vi "UHR-Fleezers Control (host) - 12.7b.vi"() -> ()   [LabVIEW 2012] (continued)
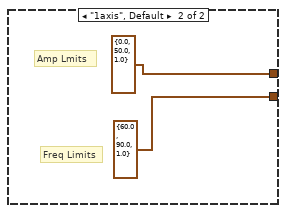
[diagram p2: hidden frame]
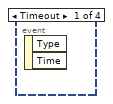
[diagram p3: hidden frame]
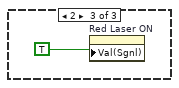
[diagram p6: hidden frame]
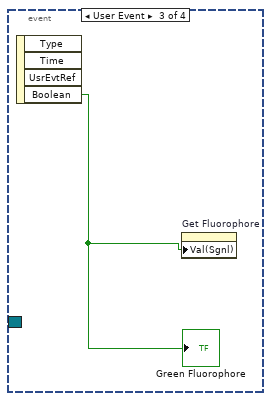
[diagram p7: hidden frame]
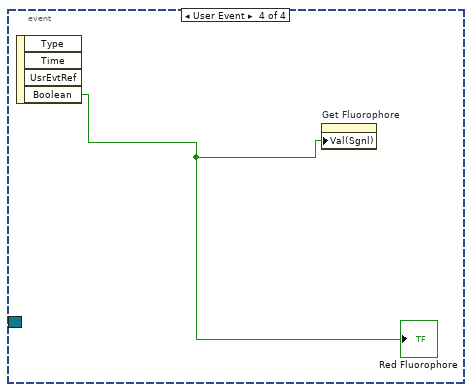
[diagram p8: hidden frame]
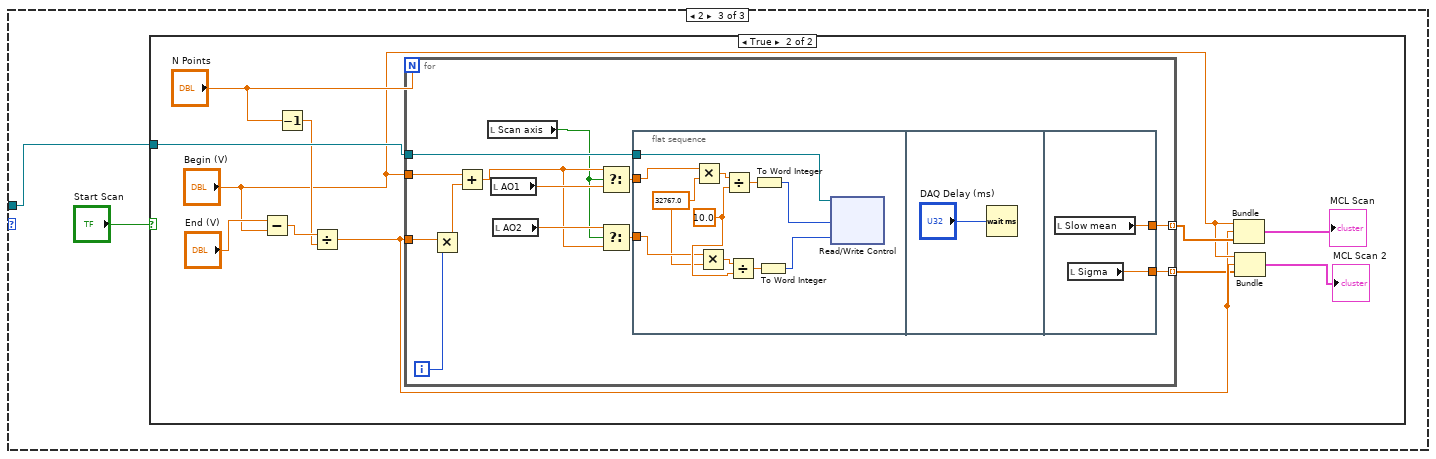
[diagram p10: hidden frame]
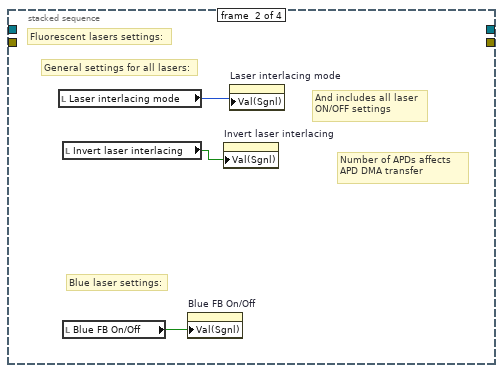
[diagram p12: hidden frame]
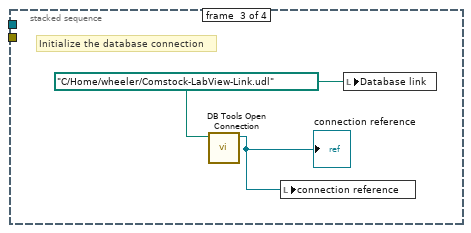
[diagram p13: hidden frame]
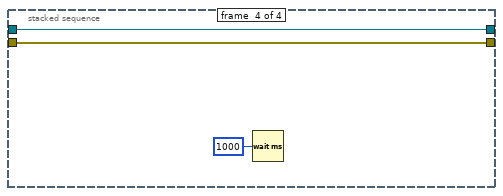
[diagram p14: hidden frame]
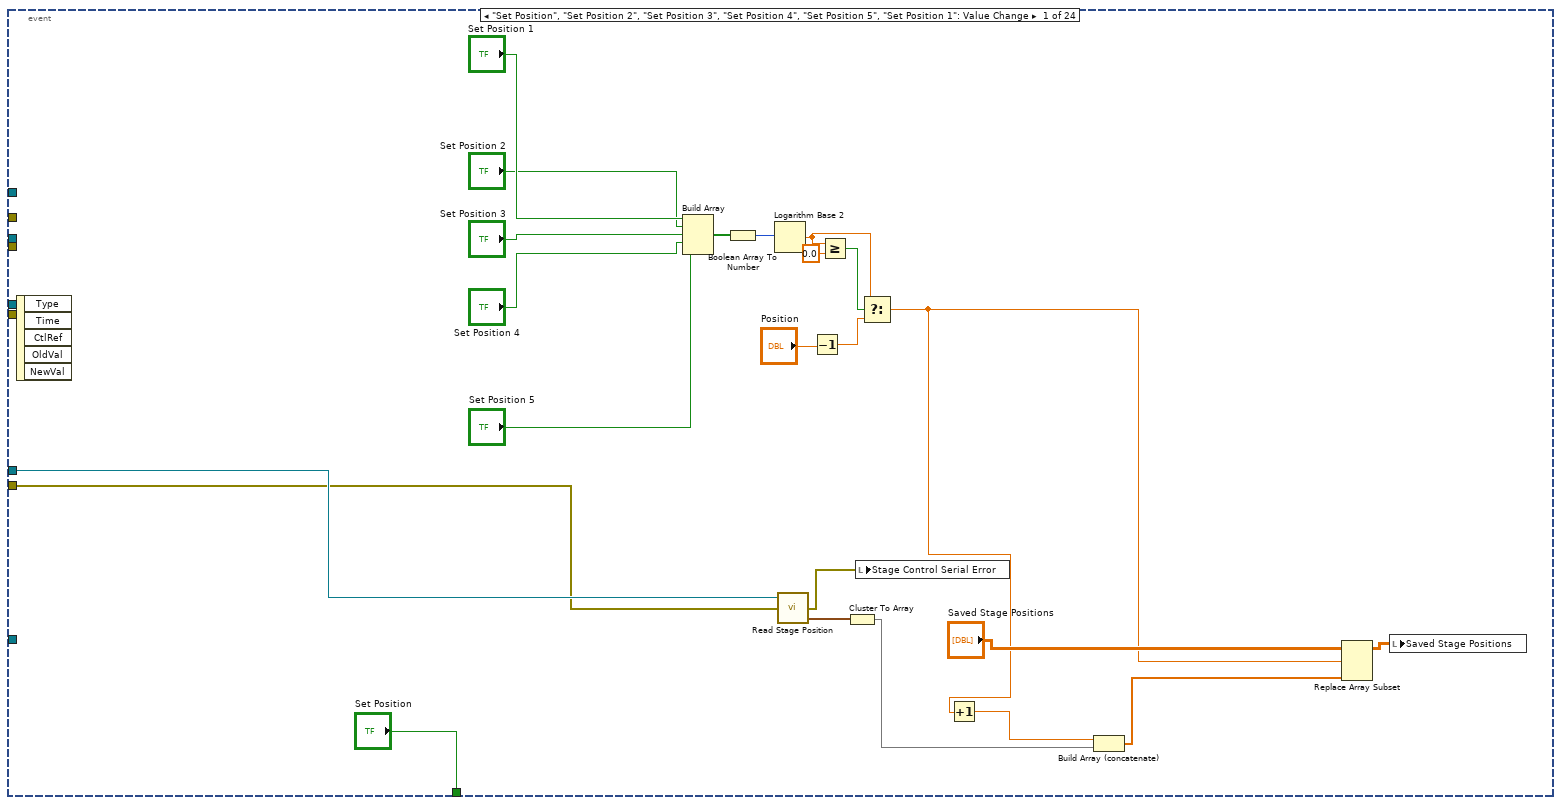
[diagram p16: hidden frame]
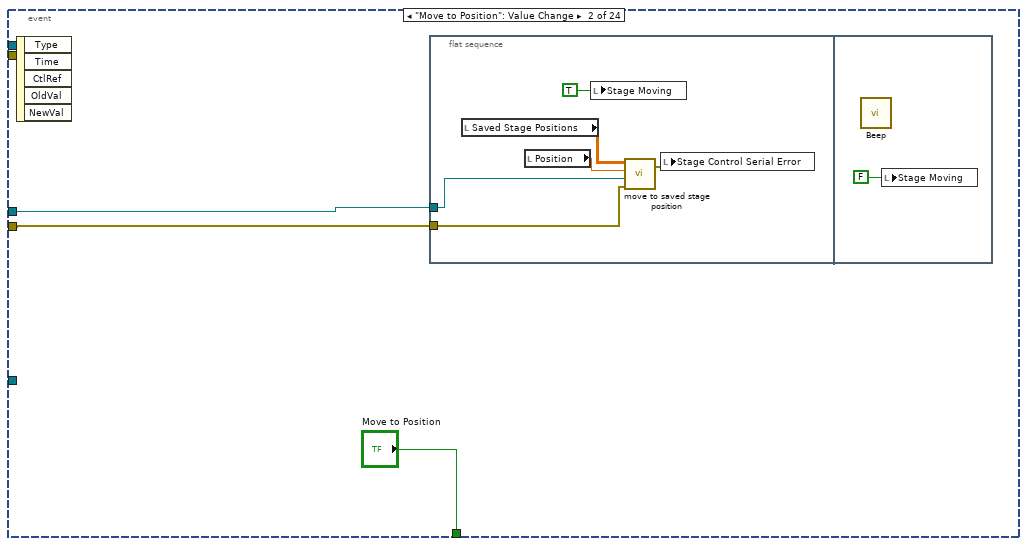
[diagram p17: hidden frame]
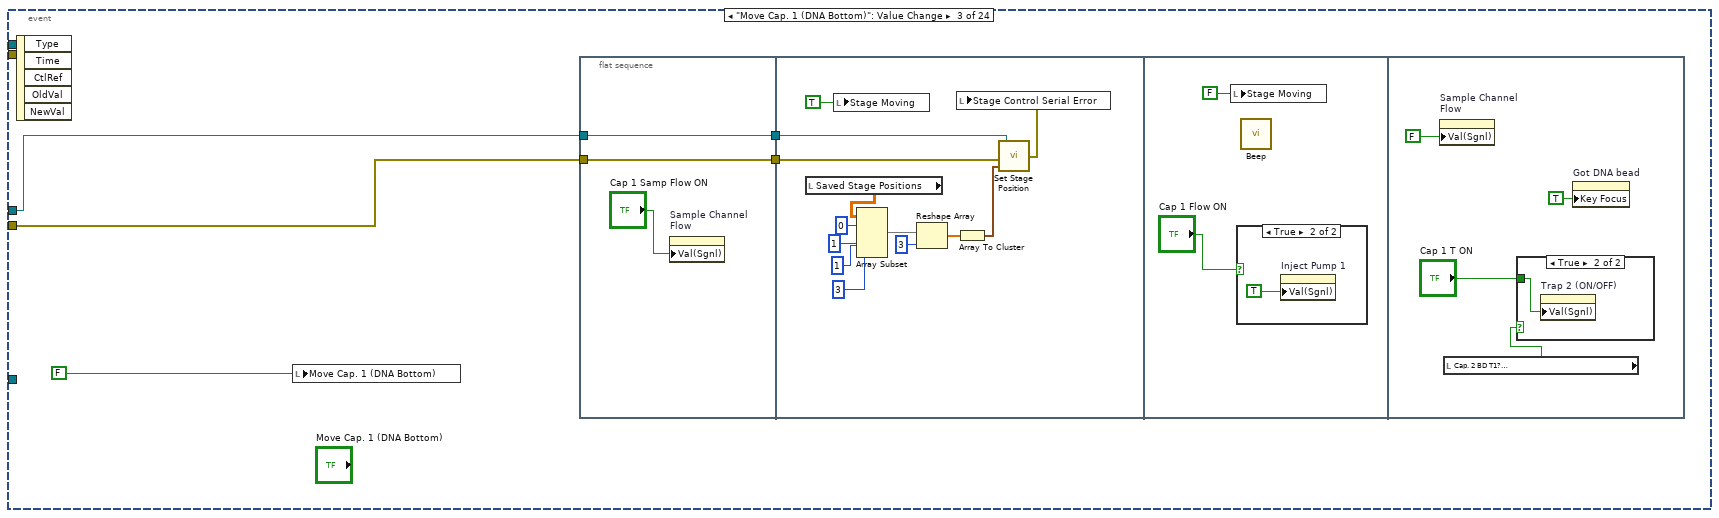
[diagram p18: hidden frame]
                n3006 = Build Array (concatenate)(w4814, w4813, w4806) -> (w4812:dbl[])
                "Calibrating Trap..." <- TRUE ("Calibrating...")
              }
              frame 4 {
                w4824 = 0.0 ("f")
                # "scan dir (x/y = 0/1)"
                # "cycles/step"
                # "n scans (f/b)"
                # "steps"
                # "freq. range"
                # "AOD raster scan"
                n3007 = local read "Number of F/B Scans (AOD)"() -> (w4831:u16)
                n3008 = local read "Cycles/step (AOD)"() -> (w4833:u64)
                n3009 = local read "Scan Range (MHz)"() -> (w4836:dbl)
                n3010 = local read "Scan steps (AOD)"() -> (w4835:u64)
                n3011 = local read "Scan BD"() -> (w4843:bool)
                n3012 = local read "Save ave N"() -> (w4848:dbl)
                n3013 = Boolean To (0,1)(Boolean=w4843) -> (0, 1=w4842:i16)
                n3014 = To Double Precision Float(number=w4831) -> (double precision float=w4830:dbl)
                n3015 = To Double Precision Float(number=w4835) -> (double precision float=w4834:dbl)
                n3016 = To Double Precision Float(number=w4833) -> (double precision float=w4832:dbl)
                n3017 = To Double Precision Float(number=w4842) -> (double precision float=w4841:dbl)
                n3018 = Multiply(x=w4848, y=w4826) -> (x*y=w4847:dbl)
                n3019 = To Double Precision Float(number=w4819) -> (double precision float=w4825:dbl)
                n3020 = Build Array(w4825, w4824, w4824, w4824, w4824) -> (w4822:dbl[])
                n3021 = local read "N sets should be saved"() -> (w4828:dbl)
                n3022 = Build Array(w4841, w4836, w4834, w4832, w4830) -> (w4838:dbl[])
                n3023 = Build Array(w4821, w4826, w4847, w4846, w4845, 2.0 ("t")) -> (w4840:dbl[])
                n3024 = Round Toward +Infinity(x=w4828) -> (ceil(x): smallest int >= x=w4829:dbl)
                n3025 = Build Array (concatenate)(w4840, w4839, w4822, w4838) -> (w4837:dbl[])
                n3026 = To Unsigned Long Integer(number=w4829) -> (unsigned 32bit integer=w4827:u32)
              }
              frame 8 {
                w4857 = 0.0 ("f")
                # "MCL raster scan"
                n3027 = local read "Number of scans (MCL)"() -> (w4852:u64)
                n3028 = local read "Scan lines (y)"() -> (w4851:u64)
                n3029 = local read "2D or 1D Scan"() -> (w4854:bool)
                n3030 = local read "Scan Range (V)\n(of steps)"() -> (w4873:dbl)
                n3031 = local read "Fast Scan Dir"() -> (w4880:bool)
                n3032 = local read "Cycles/step (MCL)"() -> (w4870:u64)
                n3033 = local read "Scan steps (MCL)"() -> (w4872:u64)
                n3034 = Select(t=w4851, s=w4854, f=w4852) -> (s? t:f=w4853:u64)
                n3035 = Boolean To (0,1)(Boolean=w4854) -> (0, 1=w4856:i16)
                n3036 = local read "Save ave N"() -> (w4885:dbl)
                n3037 = local read "Initial X"() -> (w4859:dbl)
                n3038 = local read "Initial Y"() -> (w4858:dbl)
                n3039 = To Double Precision Float(number=w4856) -> (double precision float=w4855:dbl)
                n3040 = Boolean To (0,1)(Boolean=w4880) -> (0, 1=w4879:i16)
                n3041 = To Double Precision Float(number=w4853) -> (double precision float=w4868:dbl)
                n3042 = To Double Precision Float(number=w4872) -> (double precision float=w4871:dbl)
                n3043 = To Double Precision Float(number=w4870) -> (double precision float=w4869:dbl)
                n3044 = To Double Precision Float(number=w4879) -> (double precision float=w4878:dbl)
                n3045 = Multiply(x=w4885, y=w4864) -> (x*y=w4884:dbl)
                n3046 = To Double Precision Float(number=w4849) -> (double precision float=w4863:dbl)
                n3047 = local read "N sets should be saved (MCL)"() -> (w4866:dbl)
                n3048 = Build Array(w4863, w4855, w4857, w4857, w4857) -> (w4861:dbl[])
                n3049 = Build Array(w4878, w4873, w4871, w4869, w4868, w4859, w4858) -> (w4875:dbl[])
                n3050 = Build Array(w4860, w4864, w4884, w4883, w4882, 3.0 ("t")) -> (w4877:dbl[])
                n3051 = Round Toward +Infinity(x=w4866) -> (ceil(x): smallest int >= x=w4867:dbl)
                n3052 = Build Array (concatenate)(w4877, w4876, w4861, w4875) -> (w4874:dbl[])
                n3053 = To Unsigned Long Integer(number=w4867) -> (unsigned 32bit integer=w4865:u32)
              }
            }
            n3054 = local read "Index"() -> (w4723:dbl)
            n3055 = call "Create new save file.vi"("Insert"="", "Ext"=".dat", "Index In"=w4723) -> ("Path Out"=w4679:path, "Index Out"=w4697:dbl)
            n3056 = local write "Save file name"(w4679) -> ()
            n3057 = local write "Index"(w4697) -> ()
            n3058 = local write "Save index"(w4697) -> ()
            n3059 = Array Size(array=w4706) -> (size(s)=w4707:i32)
            n3060 = Open/Create/Replace File(file path (use dialog)=w4679, operation (0:open)=T29."create", access (0:read/write)=enum16{"read/write", "read-only", "write-only"}."write-only") -> (refnum out=w4720:refnum<file>)  [unwired: 1 in, 4 out]
            n3061 = local write "Saving..."(TRUE ("Saving...")) -> ()
            n3062 = To Double Precision Float(number=w4707) -> (double precision float=w4705:dbl)
            n3063 = String Length(string="Comment (data description)") -> (length=w4704:i32)
            n3064 = To Double Precision Float(number=w4704) -> (double precision float=w4703:dbl)
            n3065 = Deny Access(7:w4720) -> (3:w4719:refnum<file>)  [unwired: 1 in, 2 out]
            n3066 = Build Array (concatenate)(w4705, w4706, w4703) -> (w4678:dbl[])
            n3067 = case "If fluorescence data to be saved" shown="True" w4695 {
              tunnel: w4679 -> [_ w4773]
              tunnel: [refnum<k0> refnum w4753] -> w4696
              frame False {
              }
              frame True {
                w4752 = 0.0
                n3068 = local read "APD Integration Time (s)"() -> (w4758:dbl)
                n3069 = local read "N APD Samp/step"() -> (w4751:dbl)
                n3070 = local read "Number of APDs"() -> (w4750:u8)
                n3071 = Path To String(path=w4773) -> (string=w4772:string)
                n3072 = String Length(string=w4772) -> (length=w4771:i32)
                n3073 = Subtract(x=w4771, y=4) -> (x-y=w4769:i32)
                n3074 = String Subset(string=w4772, length (rest)=w4769) -> (substring=w4768:string)  [unwired: 1 out]
                n3075 = Build Array(w4758, w4751, w4750, w4752, w4752, w4752, w4752, w4752) -> (w4755:dbl[])
                n3076 = Concatenate Strings(w4768, "_fl.dat" ("string")) -> (w4766:string)
                n3077 = Array Size(array=w4755) -> (size(s)=w4757:i32)
                n3078 = String To Path(string=w4766) -> (path=w4762:path)
                n3079 = Open/Create/Replace File(file path (use dialog)=w4762, operation (0:open)=T29."create", access (0:read/write)=enum16{"read/write", "read-only", "write-only"}."write-only") -> (refnum out=w4763:refnum<file>)  [unwired: 1 in, 4 out]
                n3080 = Deny Access(7:w4763) -> (3:w4759:refnum<file>)  [unwired: 1 in, 2 out]
                n3081 = To Double Precision Float(number=w4757) -> (double precision float=w4756:dbl)
                n3082 = Build Array (concatenate)(w4756, w4755) -> (w4754:dbl[])
                n3083 = Write to Binary File(file (use dialog)=w4759, data=w4754, 5:FALSE ("prepend array or string size? (T)"), 9:T28."big-endian, network order" ("byte order (0:big-endian, network order)")) -> (refnum out=w4753:refnum<file>)  [unwired: 1 in, 3 out]
              }
            }
            n3084 = case shown="True" w4683 {
              tunnel: w4679 -> [_ w4734]
              tunnel: [refnum<k0> refnum w4733] -> w4684
              frame False {
              }
              frame True {
                w4729 = 0.0 ("element")
                n3085 = Path To String(path=w4734) -> (string=w4748:string)
                n3086 = Build Array(w4729, w4729, w4729, w4729, w4729, w4729, w4729, w4729) -> (w4730:dbl[])
                n3087 = String Length(string=w4748) -> (length=w4747:i32)
                n3088 = Subtract(x=w4747, y=4) -> (x-y=w4745:i32)
                n3089 = Array Size(array=w4730) -> (size(s)=w4732:i32)
                n3090 = String Subset(string=w4748, length (rest)=w4745) -> (substring=w4744:string)  [unwired: 1 out]
                n3091 = To Double Precision Float(number=w4732) -> (double precision float=w4731:dbl)
                n3092 = Concatenate Strings(w4744, "_pos.dat" ("string")) -> (w4742:string)
                n3093 = Build Array (concatenate)(w4731, w4730) -> (w4728:dbl[])
                n3094 = String To Path(string=w4742) -> (path=w4738:path)
                n3095 = Open/Create/Replace File(file path (use dialog)=w4738, operation (0:open)=T29."create", access (0:read/write)=enum16{"read/write", "read-only", "write-only"}."write-only") -> (refnum out=w4739:refnum<file>)  [unwired: 1 in, 4 out]
                n3096 = Deny Access(7:w4739) -> (3:w4735:refnum<file>)  [unwired: 1 in, 2 out]
                n3097 = Write to Binary File(file (use dialog)=w4735, data=w4728, 5:FALSE ("prepend array or string size? (T)"), 9:T28."big-endian, network order" ("byte order (0:big-endian, network order)")) -> (refnum out=w4733:refnum<file>)  [unwired: 1 in, 3 out]
              }
            }
            n3098 = Write to Binary File(file (use dialog)=w4719, data=w4678, 5:w4701, 9:w4700) -> (refnum out=w4702:refnum<file>)  [unwired: 1 in, 3 out]
            n3099 = Write to Binary File(file (use dialog)=w4702, data="Comment (data description)", 5:w4701, 9:w4700) -> (refnum out=w4699:refnum<file>)  [unwired: 1 in, 3 out]
            n3100 = local read "connection reference"() -> (w4681:T17)
            n3101 = Bundle("Comment (data description)"="Comment (data description)", "Channel 1 Buffer"="Channel 1 Buffer", "Channel 2 Buffer"="Channel 2 Buffer", "Channel 3 Buffer"="Channel 3 Buffer", "Title"="Title", "DNA Construct"="DNA Construct", "Bead diameter"="Bead diameter", "Name"="Name") -> (w4669:T47)  [unwired: 1 in]
            n3102 = call "MattFileCreator-v9.vi"("Comments"=w4669, "Input Array"=w4678, "File path"=w4679, "table"="labview", "connection reference"=w4681) -> ("connection reference out"=w4680:T17)  [unwired: 5 in, 1 out]
            n3103 = local write "connection reference"(w4680) -> ()
          }
        }
        n3104 = feedback-in #27(w4629) -> ()
        n3105 = feedback-in #28(w4656) -> ()
        n3106 = feedback-in #29(w4628) -> ()
        n3107 = feedback-in #30(w4639) -> ()
        n3108 = feedback-in #31(w4642) -> ()
        n3109 = feedback-in #32(w4655) -> ()
        n3110 = feedback-in #33(w4645) -> ()
      }
      frame #1 {
        n3111 = local read "Saving..."() -> (w4899:bool)
        n3112 = case shown="True" w4899 {
          tunnel: w4903 -> [_ w4914]
          tunnel: w4902 -> [_ w4928]
          tunnel: w4901 -> [_ w4924]
          tunnel: w4900 -> [_ w4923]
          tunnel: w4898 -> [_ w4922]
          tunnel: w4897 -> [_ w4917]
          tunnel: w4896 -> [_ w4916]
          tunnel: w4895 -> [_ w4915]
          tunnel: w4894 -> [_ w4913]
          tunnel: w4893 -> [_ w4911]
          tunnel: w4892 -> [_ w4910]
          tunnel: w4891 -> [_ w4909]
          tunnel: w4890 -> [_ w4908]
          tunnel: w4889 -> [_ w4907]
          tunnel: w4888 -> [_ w4906]
          tunnel: w4887 -> [_ w4905]
          tunnel: w4886 -> [_ w4904]
          frame False {
          }
          frame True {
            n3113 = Multiply(x=w4914, y=w4913) -> (x*y=→"Time (s)":dbl)
            n3114 = Less Or Equal?(x=w4914, y=w4922) -> (x <= y?=w4926:bool)
            n3115 = Or(x="Stop Saving", y="Abort save 2") -> (x .or. y?=w4918:bool)
            n3116 = Not(x=w4918) -> (.not. x?=w4927:bool)
            n3117 = And(x=w4926, y=w4927) -> (x .and. y?=w4925:bool)
            n3118 = case shown="True" w4925 {
              tunnel: w4928 -> [w4935 w5026]
              tunnel: [0.0 w5029] -> w4921
              tunnel: w4914 -> [_ w5027]
              tunnel: w4922 -> [_ w5028]
              tunnel: w4924 -> [_ w5023]
              tunnel: w4923 -> [_ _]
              tunnel: w4917 -> [w4933 w5016]
              tunnel: w4916 -> [w4932 w5017]
              tunnel: w4915 -> [_ w5015]
              tunnel: w4911 -> [_ w5014]
              tunnel: w4910 -> [_ w4938]
              tunnel: w4909 -> [_ w5007]
              tunnel: w4908 -> [_ w4954]
              tunnel: w4907 -> [w4929 w4971]
              tunnel: w4906 -> [w4930 w4970]
              tunnel: w4905 -> [_ w4967]
              tunnel: w4904 -> [_ w4965]
              frame False {
                w4931 = FALSE
                n3119 = Close File(refnum=w4935) -> ()  [unwired: 1 in, 2 out]
                n3120 = case shown="True" w4932 {
                  tunnel: w4933 -> [_ w4937]
                  frame False {
                  }
                  frame True {
                    n3121 = Close File(refnum=w4937) -> ()  [unwired: 1 in, 2 out]
                  }
                }
                n3122 = case shown="True" w4929 {
                  tunnel: w4930 -> [_ w4936]
                  frame False {
                  }
                  frame True {
                    n3123 = Close File(refnum=w4936) -> ()  [unwired: 1 in, 2 out]
                  }
                }
                n3124 = local write "Raster Scanning..."(w4931) -> ()
                n3125 = local write "Calibrating Trap..."(w4931) -> ()
                n3126 = call <vilib>:"Beep.vi"() -> ()  [unwired: 3 in, 9 out]
                n3127 = local write "Stop Saving"(w4931) -> ()
                "Saving..." <- w4931
              }
              frame True {
                n3128 = local read "Calibrating Trap..."() -> (w5018:bool)
                n3129 = case "Write fl. data" shown="True" w5017 {
                  tunnel: w5016 -> [_ w5052]
                  tunnel: w5015 -> [_ w5051]
                  frame False {
                  }
                  frame True {
                    n3130 = Write to Binary File(file (use dialog)=w5052, data=w5051, 5:FALSE ("prepend array or string size? (T)"), 9:T28."big-endian, network order" ("byte order (0:big-endian, network order)")) -> ()  [unwired: 1 in, 4 out]
                  }
                }
                n3131 = Greater?(x="Save ave N", y=1.0) -> (0:w5021:bool)
                n3132 = Not(x=w5018) -> (.not. x?=w5020:bool)
                n3133 = And(x=w5020, y=w5021) -> (x .and. y?=w4968:bool)
                n3134 = case shown="True" w4968 {
                  tunnel: w4967 -> [w5032 w5043]
                  tunnel: [w5032 w5035] -> w4966
                  tunnel: "Save ave N" -> [_ w5036]
                  frame False {
                  }
                  frame True {
                    w5033 = 2 ("dimension size")
                    n3135 = Array Size(array=w5043) -> (size(s)=w5037:i32)
                    n3136 = Divide(x=w5037, y=w5033) -> (x/y=w5041:dbl)
                    n3137 = Reshape Array(w5043, w5041, w5033) -> (w5042:u64[][])
                    n3138 = Transpose 2D Array(2D array=w5042) -> (transposed array=w5040:u64[][])
                    n3139 = for {
                      tunnel: w5040 -> [w5045] mode=indexing
                      tunnel: [w5044] -> w5034 mode=indexing
                      tunnel: w5036 -> [w5046]
                      workers-P: _ -> [_]
                      n3140 = call "downsample 1D array - U64.vi"("Ave N"=w5046, "Array In"=w5045) -> ("Array Out"=w5044:u64[])  [unwired: 1 in]
                    }
                    n3141 = Transpose 2D Array(2D array=w5034) -> (transposed array=w5039:u64[][])
                    n3142 = Divide(x=w5037, y=w5036) -> (x/y=w5038:dbl)
                    n3143 = Reshape Array(w5039, w5038) -> (w5035:u64[])
                  }
                }
                n3144 = case shown="True" w4968 {
                  tunnel: w5023 -> [w5055 w5067]
                  tunnel: [w5055 w5059] -> w5019
                  tunnel: "Save ave N" -> [_ w5060]
                  tunnel: w5014 -> [_ w5058]
                  frame False {
                  }
                  frame True {
                    n3145 = Array Size(array=w5067) -> (size(s)=w5061:i32)
                    n3146 = Array Size(array=w5058) -> (size(s)=w5057:i32)
                    n3147 = Divide(x=w5061, y=w5057) -> (x/y=w5065:dbl)
                    n3148 = Reshape Array(w5067, w5065, w5057) -> (w5066:i16[][])
                    n3149 = Transpose 2D Array(2D array=w5066) -> (transposed array=w5064:i16[][])
                    n3150 = for {
                      tunnel: w5064 -> [w5070] mode=indexing
                      tunnel: [w5069] -> w5056 mode=indexing
                      tunnel: w5060 -> [w5068]
                      workers-P: _ -> [_]
                      n3151 = call "downsample 1D array - I16.vi"("Ave N"=w5068, "Array In"=w5070) -> ("Array Out"=w5069:i16[])  [unwired: 1 out]
                    }
                    n3152 = Transpose 2D Array(2D array=w5056) -> (transposed array=w5063:i16[][])
                    n3153 = Divide(x=w5061, y=w5060) -> (x/y=w5062:dbl)
                    n3154 = Reshape Array(w5063, w5062) -> (w5059:i16[])
                  }
                }
                n3155 = Index Array(array=w4954, index=2) -> (element=w4955:waveform(dbl))
                n3156 = Index Array(array=w4954, index=1) -> (element=w4988:waveform(dbl))
                n3157 = Index Array(array=w4954, index=0) -> (element=w4990:waveform(dbl))
                n3158 = Unbundle By Name(w4955) -> ("Y"=w4957:dbl[])
                n3159 = Unbundle By Name(w4988) -> ("Y"=w4992:dbl[])
                n3160 = Unbundle By Name(w4990) -> ("Y"=w5000:dbl[])
                n3161 = case "Write trap pos. data" shown="True" w4971 {
                  tunnel: w4970 -> [_ w5048]
                  tunnel: w4966 -> [_ w5047]
                  frame False {
                  }
                  frame True {
                    n3162 = Write to Binary File(file (use dialog)=w5048, data=w5047, 5:FALSE ("prepend array or string size? (T)"), 9:T28."big-endian, network order" ("byte order (0:big-endian, network order)")) -> ()  [unwired: 1 in, 4 out]
                  }
                }
                n3163 = Write to Binary File(file (use dialog)=w5026, data=w5019, 5:FALSE ("prepend array or string size? (T)"), 9:T28."big-endian, network order" ("byte order (0:big-endian, network order)")) -> ()  [unwired: 1 in, 4 out]
                n3164 = feedback #34(w4957) -> (w4958:dbl[])
                n3165 = Build Array (concatenate)(w4958, w4957) -> (w4953:dbl[])
                n3166 = Select(t=w4957, s=w4938, f=w4953) -> (s? t:f=w4943:dbl[])
                n3167 = feedback-in #34(w4943) -> ()
                n3168 = feedback #35(w4992) -> (w4994:dbl[])
                n3169 = Build Array (concatenate)(w4994, w4992) -> (w4993:dbl[])
                n3170 = Select(t=w4992, s=w4938, f=w4993) -> (s? t:f=w4982:dbl[])
                n3171 = feedback-in #35(w4982) -> ()
                n3172 = feedback #36(w5000) -> (w5013:dbl[])
                n3173 = Build Array (concatenate)(w5013, w5000) -> (w5012:dbl[])
                n3174 = Select(t=w5000, s=w4938, f=w5012) -> (s? t:f=w4987:dbl[])
                n3175 = feedback-in #36(w4987) -> ()
                n3176 = Divide(x=w5027, y=w5028) -> (x/y=w5030:dbl)
                n3177 = Multiply(x=w5030, y=100.0) -> (x*y=w5029:dbl)
                n3178 = Build Array(w4987, w4982, w4943) -> (→"Saved APD":dbl[][])
                n3179 = Array Size(array=w4987) -> (size(s)=w5005:i32)
                n3180 = Unbundle By Name(w5007) -> ("Y"=w5011:dbl[])
                n3181 = Subtract(x=w5005, y="N pts to average") -> (x-y=w4940:i32)
                n3182 = Multiply(x="N pts to average", y=u16 2) -> (x*y=w4983:u16)
                n3183 = Subtract(x=w5005, y=w4983) -> (x-y=w4941:i32)
                n3184 = feedback #37(w5011) -> (w5010:dbl[])
                n3185 = Build Array (concatenate)(w5010, w5011) -> (w5009:dbl[])
                n3186 = Select(t=w5011, s=w4938, f=w5009) -> (s? t:f=w5008:dbl[])
                "Trap Delta Graph" <- w5008
                n3187 = feedback-in #37(w5008) -> ()
                n3188 = Array Subset(array=w4987, index=w4940, length="N pts to average") -> (w5004:dbl[])
                n3189 = Array Subset(array=w4987, index=w4941, length="N pts to average") -> (w5003:dbl[])
                n3190 = Array Subset(array=w4982, index=w4940, length="N pts to average") -> (w4985:dbl[])
                n3191 = Array Subset(array=w4982, index=w4941, length="N pts to average") -> (w4984:dbl[])
                n3192 = Array Subset(array=w4943, index=w4940, length="N pts to average") -> (w4952:dbl[])
                n3193 = Array Subset(array=w4943, index=w4941, length="N pts to average") -> (w4951:dbl[])
                n3194 = Index Array(array=w4965, index=0) -> (element=w4963:waveform(dbl))
                n3195 = call-poly <vilib>:"Mean.vi"("X"=w5004) -> ("mean"=w5002:dbl)  [unwired: 1 out]
                n3196 = call-poly <vilib>:"Mean.vi"("X"=w4985) -> ("mean"=w4981:dbl)  [unwired: 1 out]
                n3197 = call-poly <vilib>:"Mean.vi"("X"=w5003) -> ("mean"=w5001:dbl)  [unwired: 1 out]
                n3198 = call-poly <vilib>:"Mean.vi"("X"=w4984) -> ("mean"=w4980:dbl)  [unwired: 1 out]
                n3199 = call-poly <vilib>:"Mean.vi"("X"=w4952) -> ("mean"=w4950:dbl)  [unwired: 1 out]
                n3200 = call-poly <vilib>:"Mean.vi"("X"=w4951) -> ("mean"=w4949:dbl)  [unwired: 1 out]
                n3201 = Unbundle By Name(w4963) -> ("Y"=w4961:dbl[])
                n3202 = Subtract(x=w4981, y=w4980) -> (x-y=w4972:dbl)
                "Delta Fl. 2" <- w4972
                n3203 = Subtract(x=w4950, y=w4949) -> (x-y=w4944:dbl)
                "Delta Fl. 3" <- w4944
                n3204 = Subtract(x=w5002, y=w5001) -> (x-y=w4999:dbl)
                "Delta Fl. 1" <- w4999
                n3205 = feedback #38(w4961) -> (w4960:dbl[])
                n3206 = Build Array (concatenate)(w4960, w4961) -> (w4962:dbl[])
                n3207 = Initialize Array(w4999, 1 ("dimension size")) -> (w4996:dbl[])
                n3208 = Initialize Array(w4972, 1 ("dimension size")) -> (w4977:dbl[])
                n3209 = Initialize Array(w4944, 1 ("dimension size")) -> (w4946:dbl[])
                n3210 = Select(t=w4961, s=w4938, f=w4962) -> (s? t:f=w4959:dbl[])
                "Saved trap pos" <- w4959
                n3211 = feedback-in #38(w4959) -> ()
                n3212 = feedback #39(w4996) -> (w4997:dbl[])
                n3213 = Build Array (concatenate)(w4997, w4996) -> (w4995:dbl[])
                n3214 = feedback #40(w4977) -> (w4978:dbl[])
                n3215 = feedback #41(w4946) -> (w4947:dbl[])
                n3216 = Build Array (concatenate)(w4978, w4977) -> (w4976:dbl[])
                n3217 = Build Array (concatenate)(w4947, w4946) -> (w4945:dbl[])
                n3218 = Select(t=w4996, s=w4938, f=w4995) -> (s? t:f=w4975:dbl[])
                n3219 = feedback-in #39(w4975) -> ()
                n3220 = Select(t=w4977, s=w4938, f=w4976) -> (s? t:f=w4974:dbl[])
                n3221 = feedback-in #40(w4974) -> ()
                n3222 = Select(t=w4946, s=w4938, f=w4945) -> (s? t:f=w4939:dbl[])
                n3223 = feedback-in #41(w4939) -> ()
                n3224 = Build Array(w4975, w4974, w4939) -> (→"Save APD Deriv":dbl[][])
              }
            }
            "Progress" <- w4921
            "Progress 2" <- w4921
          }
        }
      }
    }
    n3225 = local read "wait to reset values"() -> (w3573:bool)
    n3226 = Not(x=w3571) -> (.not. x?=w3574:bool)
    n3227 = And(x=w3574, y=w3573) -> (x .and. y?=w3575:bool)
    n3228 = case "Part of MCL raster scanning: returns to initial positions after scan done" shown="True" w3575 {
      tunnel: w3306 -> [w4449 w4456]
      tunnel: [w4449 w4455] -> w3577
      tunnel: w3305 -> [w4448 w4454]
      tunnel: [w4448 w4453] -> w3572
      frame False {
      }
      frame True {
        w4464 = 10.0 ("y")
        w4463 = 32767.0 ("y")
        # "to return scan values\nafter a synchronous \nAOM scan"
        n3229 = local read "AO2"() -> (w4457:dbl)
        n3230 = local read "AO1"() -> (w4458:dbl)
        n3231 = local write "wait to reset values"(FALSE ("wait to reset values")) -> ()
        n3232 = Multiply(x=w4458, y=w4463) -> (x*y=w4460:dbl)
        n3233 = Multiply(x=w4457, y=w4463) -> (x*y=w4462:dbl)
        n3234 = Divide(x=w4460, y=w4464) -> (x/y=w4459:dbl)
        n3235 = Divide(x=w4462, y=w4464) -> (x/y=w4461:dbl)
        n3236 = To Word Integer(number=w4459) -> (16bit integer=w4465:i16)
        n3237 = To Word Integer(number=w4461) -> (16bit integer=w4466:i16)
        n3238 = local read "Total Counts (ticks)"() -> (w4450:u16)
        n3239 = xnode "Read/Write Control"("FPGA VI Reference In"=w4456, "error in"=w4454, "AO1"=w4465, "AO2"=w4466, "MCL count"=w4450) -> ("FPGA VI Reference Out"=w4455:T20, "error out"=w4453:errorcluster)
        n3240 = local read "Scan Range (V)\n(of steps)"() -> (w4451:dbl)
        n3241 = property on="Scan Range (V)\n(of steps)" class="DigNum (strict)"("Val(Sgnl)"=w4451) -> ()  [unwired: 2 in, 2 out]
      }
    }
    n3242 = node-c288() -> ()  [unwired: 2 out]
  }
  n3243 = flat-sequence "Video" {
    tunnel: [w5080] -> w121
    tunnel: w121 -> [w5120]
    frame #0 {
      n3244 = while {
        stop <- w5072 continue-if-true
        n3245 = call "Close Video Capture.vi"() -> ("error code OUT"=w5074:i32)
        n3246 = Equal?(x=w5074, y=0) -> (x = y?=w5072:bool)
      }
      n3247 = local write "Stop All"(FALSE ("Stop All")) -> ()
    }
    frame #1 {
      n3248 = call "DMR_Init.vi"() -> ()  [unwired: 3 out]
    }
    frame #2 {
      w5075 = "DE245428202"  # MSU fleezers card #
      (unwired) "DE019116701"  # Illinois fleezers card #
      # "Setting the destination format to Mono8 makes sure that the image can be displayed in the intensity plot."
      n3249 = call "DMR_GetDevice.vi"("search string IN"=w5075) -> ("device handle OUT"=w5098:i32)  [unwired: 4 in, 2 out]
      n3250 = call "DMR_OpenDevice.vi"("device handle IN"=w5098) -> ("driver handle OUT"=w5081:i32)  [unwired: 4 out]
      n3251 = call "DMR_FindList.vi"("flags IN"=u32 0 ("flags"), "list name IN"="" ("String"), "list type IN"=T48."camera descriptions", "driver handle IN"=w5081) -> ("list handle OUT"=w5084:i32)  [unwired: 2 out]
      n3252 = call "DMR_FindList.vi"("flags IN"=u32 0 ("flags"), "list name IN"="Base", "list type IN"=T48."setting", "driver handle IN"=w5081) -> ("list handle OUT"=w5082:i32)  [unwired: 2 out]
      n3253 = call "OBJ_GetHandle.vi"("object name IN"="VideoStandard", "list handle IN"=w5084) -> ("object handle OUT"=w5078:i32)  [unwired: 3 out]
      n3254 = call "OBJ_GetHandle.vi"("object name IN"="PixelFormat", "list handle IN"=w5082) -> ("object handle OUT"=w5092:i32)  [unwired: 3 out]
      n3255 = call "OBJ_SetS.vi"("value index IN"=0, "value IN"="NTSC M", "object handle IN"=w5078) -> ()  [unwired: 2 out]
      n3256 = call "OBJ_SetS.vi"("value index IN"=0, "value IN"="Mono8" ("value"), "object handle IN"=w5092) -> ()  [unwired: 2 out]
      n3257 = call "OBJ_GetHandle.vi"("object name IN"="VideoChannel", "list handle IN"=w5082) -> ("object handle OUT"=w5088:i32)  [unwired: 3 out]
      n3258 = while {
        tunnel: [w5102] -> w5080
        tunnel: w5081 -> [w5099]
        stop <- w5100 continue-if-true
        n3259 = call "DMR_ImageRequestSingle.vi"("request control IN"=0, "driver handle IN"=w5099) -> ("error code OUT"=w5101:i32, "driver handle OUT"=w5102:i32)  [unwired: 2 out]
        n3260 = Equal To 0?(x=w5101) -> (x = 0?=w5100:bool)
      }
      n3261 = call "OBJ_SetI.vi"("value index IN"=0, "value IN"=3 ("Video channel"), "object handle IN"=w5088) -> ()  [unwired: 2 out]
    }
    frame #3 {
      w5108 = T18 0 items=["Grayscale (U8)", "Grayscale (I16)", "Grayscale (SGL)", "Complex (CSG)", "RGB (U32)", "HSL (U32)", "RGB (U64)"] ("Image Type")
      w5116 = T18 0 items=["Grayscale (U8)", "Grayscale (I16)", "Grayscale (SGL)", "Complex (CSG)", "RGB (U32)", "HSL (U32)", "RGB (U64)"] ("Image Type")
      n3262 = for "Create Greyscale map" {
        N: 256 -> [_]
        tunnel: [w5122] -> w5105 mode=indexing
        workers-P: _ -> [_]
        i -> [w5125]
        n3263 = To Unsigned Byte Integer(number=w5125) -> (unsigned 8bit integer=w5121:u8)
        n3264 = Join Numbers(hi=w5121, lo=w5121) -> ((hi.lo)=w5124:u16)
        n3265 = Join Numbers(hi=w5121, lo=w5121) -> ((hi.lo)=w5123:u16)
        n3266 = Join Numbers(hi=w5124, lo=w5123) -> ((hi.lo)=w5122:u32)
      }
      n3267 = call "IMAQ Create"("Image Name"="Scaled video", "Image Type"=w5108) -> ("New Image"=w5107:T2)  [unwired: 2 in, 2 out]
      n3268 = call "IMAQ Create"("Image Name"="Main video", "Image Type"=w5116) -> ("New Image"=w5117:T2)  [unwired: 2 in, 2 out]
      n3269 = node-c288(0 ("Processor")) -> (w5115:T23)  [unwired: 3 out]
      n3270 = Initialize Array(u32 0 ("Window Number (0...15)"), 480 ("dimension size"), 640 ("dimension size")) -> (w5110:u32[][])
      n3271 = timed-loop {
        tunnel: w5120 -> [w5142]
        tunnel: [w5141] -> w5119
        tunnel: w5117 -> [w5140]
        timing: w5115 -> [_]
        timing-out: [_] -> w5114
        tunnel: w5110 -> [w5129]
        tunnel: w5107 -> [w5127]
        tunnel: w5105 -> [w5126]
        stop <- w5128 stop-if-true
        # "This block performs the \nactual image capture."
        n3272 = node-c288() -> ()  [unwired: 2 out]
        n3273 = local read "Stop All"() -> (w5128:bool)
        n3274 = Reciprocal(x="Video Capture Rate (Hz)") -> (1/x=w5132:dbl)
        n3275 = Multiply(x=w5132, y=1000.0) -> (x*y=w5130:dbl)
        n3276 = call "DMR_ImageRequestWaitFor.vi"("queue number IN"=0, "timeout(ms) IN"=500, "driver handle IN"=w5142) -> ("error code OUT"=w5146:i32, "request number OUT"=w5143:i32, "driver handle OUT"=w5144:i32)
        n3277 = feedback #42(T49 refnum ("Avi Refnum")) -> (w5134:T49)
        n3278 = case shown="True" "New Video File" {
          tunnel: [T49 refnum ("Avi Refnum") w5163] -> w5136
          tunnel: [FALSE TRUE] -> w5137
          tunnel: w5134 -> [_ w5159]
          frame False {
          }
          frame True {
            n3279 = call "Create new save file.vi"("Ext"=".avi" ("string"), "Index In"="Video Index") -> ("Path Out"=w5155:path, "Index Out"=w5156:dbl)  [unwired: 1 in]
            "Path Out" <- w5155
            n3280 = Not Equal?(x=w5159, y=T49 refnum ("Avi Refnum")) -> (x != y?=w5160:bool)
            n3281 = Increment(x=w5156) -> (x+1=w5165:dbl)
            n3282 = case shown="True" w5160 {
              tunnel: w5159 -> [_ w5166]
              frame False {
              }
              frame True {
                n3283 = call "IMAQ AVI Close"("Avi Refnum"=w5166) -> ()  [unwired: 1 in, 10 out]
              }
            }
            n3284 = local write "Video Index"(w5165) -> ()
            n3285 = call "IMAQ AVI Create"("Frames Per Second"=u32 30, "AVI Path"=w5155) -> ("Avi Refnum"=w5163:T49)  [unwired: 5 in, 4 out]
          }
        }
        n3286 = Equal To 0?(x=w5146) -> (x = 0?=w5145:bool)
        n3287 = Select(t=w5136, s=w5137, f=w5134) -> (s? t:f=w5135:T49)
        n3288 = feedback-in #42(w5135) -> ()
        n3289 = case shown="True" w5145 {
          tunnel: w5144 -> [w5167 w5201]
          tunnel: w5143 -> [_ w5200]
          tunnel: [w5167 w5197] -> w5141
          tunnel: w5140 -> [_ w5182]
          tunnel: w5129 -> [_ w5186]
          tunnel: w5135 -> [_ w5184]
          tunnel: w5127 -> [_ w5179]
          tunnel: w5126 -> [_ w5178]
          frame False {
          }
          frame True {
            w5191 = u32 0 ("X-offset IN")
            n3290 = call "DMR_GetImageRequestBufferData.vi"("driver handle IN"=w5201, "request number IN"=w5200) -> ("width OUT"=w5190:i32, "height OUT"=w5189:i32, "driver handle OUT"=w5196:i32, "request number OUT"=w5195:i32, "bytes per pixel OUT"=w5192:i32)  [unwired: 13 out]
            n3291 = call "DMR_GetImageRequestBufferImageData.vi"("driver handle IN"=w5196, "request number IN"=w5195, "bytes per pixel IN"=w5192, "X-offset IN"=w5191, "Y-offset IN"=w5191, "height IN"=w5189, "width IN"=w5190) -> ("driver handle OUT"=w5194:u32, "request number OUT"=w5193:u32, "image OUT"=w5171:u32[][])  [unwired: 10 out]
            n3292 = Transpose 2D Array(2D array=w5171) -> (transposed array=w5177:u32[][])
            n3293 = Select(t=w5177, s="Flip Y (or X)", f=w5171) -> (s? t:f=w5176:u32[][])
            n3294 = call "DMR_ImageRequestUnlock.vi"("request number IN"=w5193, "driver handle IN"=w5194) -> ("driver handle OUT"=w5199:i32)  [unwired: 1 in, 2 out]
            n3295 = for {
              tunnel: w5176 -> [w5236] mode=indexing
              tunnel: [w5235] -> w5174 mode=indexing
              n3296 = Reverse 1D Array(array=w5236) -> (reversed array=w5235:u32[])
            }
            n3297 = call "DMR_ImageRequestSingle.vi"("request control IN"=0, "driver handle IN"=w5199) -> ("driver handle OUT"=w5197:i32)  [unwired: 3 out]
            n3298 = Transpose 2D Array(2D array=w5174) -> (transposed array=w5175:u32[][])
            n3299 = Select(t=w5175, s="Flip Y (or X)", f=w5174) -> (s? t:f=w5172:u32[][])
            n3300 = Select(t=w5172, s="Flip Image", f=w5171) -> (s? t:f=w5169:u32[][])
            n3301 = case shown="True" "Averaging" {
              tunnel: w5169 -> [w5239 w5244]
              tunnel: [w5239 w5243] -> w5183
              tunnel: w5186 -> [_ w5241]
              frame False {
              }
              frame True {
                (unwired) 1
                w5249 = 1
                n3302 = feedback #43(w5241) -> (w5240:u32[][])
                n3303 = Add(x=w5244, y=w5240) -> (x+y=w5245:u32[][])
                n3304 = Select(t=w5241, s="Reset Averaging", f=w5245) -> (s? t:f=w5247:u32[][])
                n3305 = feedback-in #43(w5247) -> ()
                n3306 = feedback #44(w5249) -> (w5242:i32)
                n3307 = Divide(x=w5245, y=w5242) -> (x/y=w5246:dbl[][])
                n3308 = Increment(x=w5242) -> (x+1=w5250:i32)
                n3309 = To Unsigned Long Integer(number=w5246) -> (unsigned 32bit integer=w5243:u32[][])
                n3310 = Select(t=w5249, s="Reset Averaging", f=w5250) -> (s? t:f=w5248:i32)
                n3311 = feedback-in #44(w5248) -> ()
              }
            }
            n3312 = case shown="True" "Zoom video window" {
              tunnel: w5183 -> [_ w5215]
              tunnel: w5179 -> [_ w5214]
              frame False {
              }
              frame True {
                n3313 = To Double Precision Float(number=w5215) -> (double precision float=w5212:dbl[][])
                n3314 = In Range and Coerce(upper limit="Intensity Upper", x=w5212, lower limit="Intensity Lower") -> (coerced(x)=w5211:dbl[][])  [unwired: 1 out]
                n3315 = Subtract(x="Intensity Upper", y="Intensity Lower") -> (x-y=w5208:dbl)
                n3316 = Subtract(x=w5211, y="Intensity Lower") -> (x-y=w5209:dbl[][])
                n3317 = Divide(x=w5209, y=w5208) -> (x/y=w5210:dbl[][])
                n3318 = Multiply(x=255.0, y=w5210) -> (x*y=w5206:dbl[][])
                n3319 = To Unsigned Byte Integer(number=w5206) -> (unsigned 8bit integer=w5213:u8[][])
                n3320 = call "IMAQ ArrayToImage"("Image Pixels (U8)"=w5213, "Image"=w5214) -> ("Image Out"=w5202:T2)  [unwired: 4 in, 5 out]
                n3321 = First Call?() -> (First Call?: T/F=w5203:bool)
                n3322 = case shown="True" w5203 {
                  tunnel: w5202 -> [w5216 w5227]
                  frame False {
                    n3323 = flat-sequence {
                      tunnel: w5216 -> [w5222]
                      frame #0 {
                        w5219 = FALSE ("Get/Set Status? (Set)")
                        w5218 = 0 ("Window Number (0...15)")
                        n3324 = call "IMAQ WindSize"("Get/Set Status? (Set)"=w5219, "Window Number"=w5218) -> ("Width & Height out"=→"Window Size":cluster{"Width":i32, "Height":i32})  [unwired: 4 in, 2 out]
                        n3325 = call "IMAQ WindMove"("Window Number (0...15)"=w5218, "Get/Set Status? (Set)"=w5219) -> ("Coordinates (screen)"=→"Window Position":cluster{"X Position":i32, "Y Position":i32})  [unwired: 3 in, 1 out]
                        n3326 = call "IMAQ WindDraw"("Resize to Image Size? (Y)"=FALSE, "Window Number (0...15)"=w5218, "Image"=w5222) -> ()  [unwired: 7 in, 2 out]
                      }
                      frame #1 {
                        n3327 = call "IMAQ WindZoom 2"("Center Point"="Center Point", "Zoom to Fit? (False)"=FALSE, "Zoom Factor"="Zoom Factor") -> ()  [unwired: 5 in, 4 out]
                      }
                    }
                  }
                  frame True {
                    n3328 = flat-sequence {
                      tunnel: w5227 -> [w5230]
                      tunnel: [w5228] -> w5226
                      tunnel: w5226 -> [w5232]
                      frame #0 {
                        w5229 = TRUE ("Resize to Image Size? (Y)")
                        w5228 = 0 ("Window Number (0...15)")
                        n3329 = call "IMAQ WindNonTearing"("Window Number"=w5228, "NonTearing? (True)"=w5229) -> ()  [unwired: 8 in, 2 out]
                        n3330 = call "IMAQ WindDraw"("Resize to Image Size? (Y)"=w5229, "Window Number (0...15)"=w5228, "Image"=w5230) -> ()  [unwired: 7 in, 2 out]
                      }
                      frame #1 {
                        n3331 = call "IMAQ WindSize"("Scrollbars? (N)"=FALSE, "Width & Height"="Initial Window Size", "Window Number"=w5232) -> ()  [unwired: 3 in, 3 out]
                        n3332 = call "IMAQ WindMove"("Window Number (0...15)"=w5232, "Coordinates (screen)"="Initial Window Position") -> ()  [unwired: 3 in, 2 out]
                      }
                    }
                  }
                }
              }
            }
            n3333 = To Unsigned Byte Integer(number=w5183) -> (unsigned 8bit integer=w5181:u8[][])
            n3334 = call "IMAQ ArrayToImage"("Image Pixels (U8)"=w5181, "Image"=w5182) -> ("Image Out"=w5180:T2)  [unwired: 4 in, 5 out]
            "Primary Video Display" <- w5180
            n3335 = case shown="True" "Save Video" {
              tunnel: w5184 -> [_ w5238]
              tunnel: w5180 -> [_ w5237]
              frame False {
              }
              frame True {
                n3336 = call "IMAQ AVI Write Frame"("Image"=w5237, "Avi Refnum"=w5238) -> ()  [unwired: 2 in, 8 out]
              }
            }
            n3337 = case shown="True" "Save Image" {
              tunnel: w5181 -> [_ w5253]
              tunnel: w5178 -> [_ w5252]
              frame False {
              }
              frame True {
                n3338 = call <vilib>:"Flatten Pixmap.vi"("colors"=w5252, "8-bit pixmap"=w5253) -> ("image data"=w5259:T50)  [unwired: 4 in, 5 out]
                n3339 = call "Create new save file.vi"("Insert"="video_frame_" ("string"), "Ext"=".bmp" ("string"), "Index In"="Image Index") -> ("Path Out"=w5255:path, "Index Out"=w5260:dbl)
                n3340 = Increment(x=w5260) -> (x+1=w5254:dbl)
                n3341 = local write "Image Index"(w5254) -> ()
                n3342 = call <vilib>:"Write BMP File.vi"("image data"=w5259, "path to BMP file"=w5255) -> ()  [unwired: 1 in, 9 out]
              }
            }
          }
        }
        n3343 = node-c288(w5130) -> ()  [unwired: 1 out]
      }
      n3344 = node-c288(w5114) -> ()  [unwired: 1 out]
      n3345 = call "DMR_CloseDevice.vi"("driver handle IN"=w5119) -> ()  [unwired: 1 in, 4 out]
    }
    frame #4 {
      n3346 = call "DMR_Close.vi"() -> ()  [unwired: 1 out]
    }
  }
  n3347 = node-c288(w16) -> ()  [unwired: 1 out]
  n3348 = node-c288(w132) -> ()  [unwired: 1 out]
  n3349 = node-c288(w134) -> ()  [unwired: 1 out]
  n3350 = property on="Saved trap pos" class="WFGraph (strict)"("Visible"=FALSE) -> ()  [unwired: 2 in, 2 out]
  n3351 = property on="Trap Delta Graph" class="WFGraph (strict)"("Visible"=TRUE) -> ()  [unwired: 2 in, 2 out]
  n3352 = node-c288(w119) -> ()  [unwired: 1 out]
  n3353 = local write "Trap pos"(FALSE ("Trap pos")) -> ()
  n3354 = disable-structure shown="Disabled" {
    disable-tunnel: w123 -> [w5266 _]
    disable-tunnel: w122 -> [w5265 _]
    frame Disabled {
      n3355 = VISA Close(VISA resource name=w5266, error in (no error)=w5265) -> (error out=w5267:errorcluster)
      n3356 = call <vilib>:"Simple Error Handler.vi"("error in (no error)"=w5267) -> ()  [unwired: 1 in, 8 out]
    }
    frame Enabled {
    }
  }
  n3357 = node-c288(w130) -> ()  [unwired: 1 out]
  n3358 = node-c288(w205) -> ()  [unwired: 1 out]
  n3359 = flat-sequence {
    tunnel: w296 -> [w5271]
    tunnel: w298 -> [w5272]
    tunnel: [w5270] -> w277
    tunnel: [w5269] -> w276
    tunnel: w261 -> [_]
    tunnel: w213 -> [_]
    tunnel: w136 -> [_]
    tunnel: w277 -> [w5273]
    tunnel: w276 -> [w5274]
    frame #0 {
      w5268 = FALSE ("AI to FIFO")
      n3360 = xnode "Read/Write Control"("FPGA VI Reference In"=w5272, "error in"=w5271, "AI to FIFO"=w5268, "APD to FIFO"=w5268) -> ("FPGA VI Reference Out"=w5270:T20, "error out"=w5269:errorcluster)
    }
    frame #1 {
      n3361 = xnode "Close FPGA VI Reference"("FPGA VI Reference In"=w5273, "error in"=w5274) -> ("error out"=→"error out":errorcluster)
    }
  }
